vi "BuildThermomechanicalStave-Old.vi"() -> ()   [LabVIEW 2016] (continued)
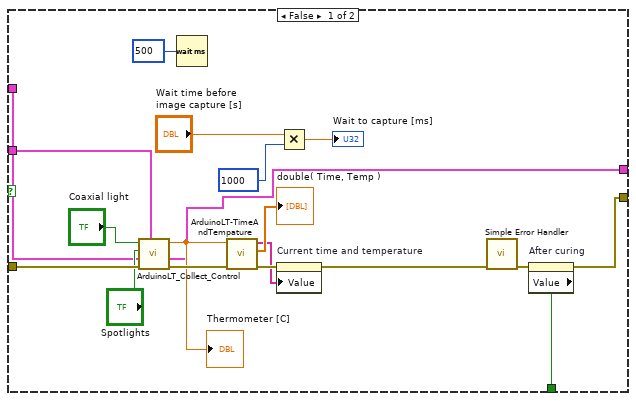
[diagram p3: hidden frame]
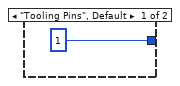
[diagram p4: hidden frame]
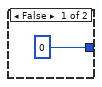
[diagram p5: hidden frame]
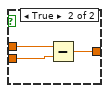
[diagram p9: hidden frame]
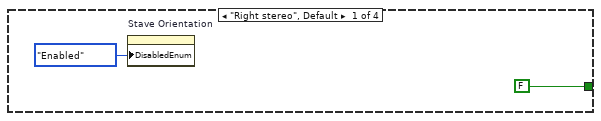
[diagram p10: hidden frame]
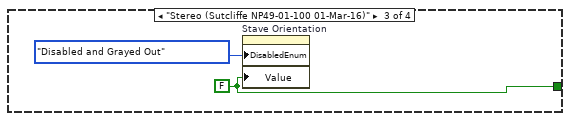
[diagram p11: hidden frame]
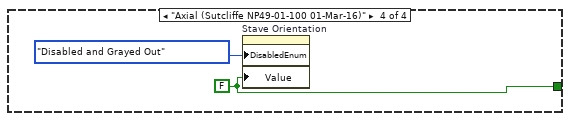
[diagram p12: hidden frame]
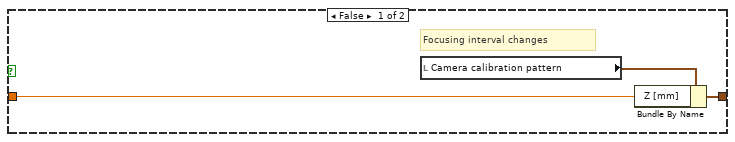
[diagram p16: hidden frame]
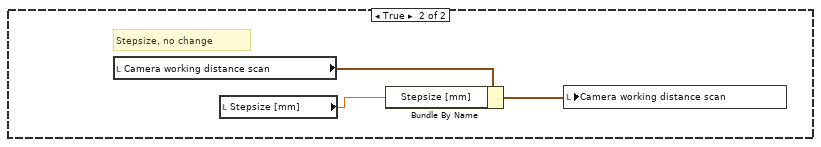
[diagram p17: hidden frame]
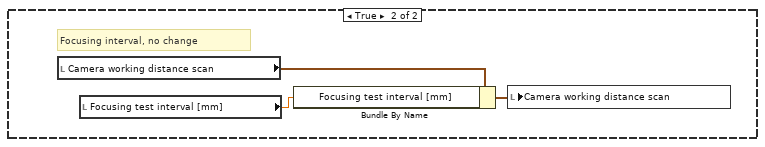
[diagram p18: hidden frame]
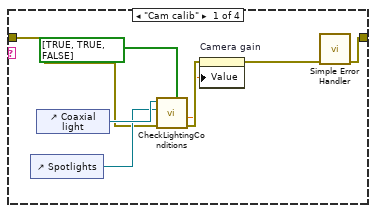
[diagram p19: hidden frame]
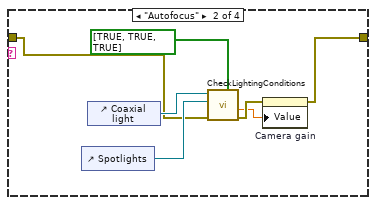
[diagram p20: hidden frame]
      n159 = Unbundle By Name("Jogging Controls") -> ("Jog step size"=w461:T16)
      n160 = control-ref of="Left"() -> (w468:refnum<vi>)
      n161 = control-ref of="Forward"() -> (w457:refnum<vi>)
      n162 = control-ref of="Up"() -> (w459:refnum<vi>)
      n163 = control-ref of="Right"() -> (w467:refnum<vi>)
      n164 = control-ref of="Backward"() -> (w456:refnum<vi>)
      n165 = call "JogStepInterpeter (SubVI).vi"("Jog step size ENUM"=w461) -> ("Jog step size"=w460:T37)
      n166 = call "ActivateToggleControls (SubVI).vi"("Left refnum"=w468, "Current stage position [mm]"=w464, "Right refnum"=w467, "Forward refnum"=w457, "Backward refnum"=w456, "error in (no error)"=w462, "Jog step size"=w460, "Up refnum"=w459, "Down refnum"=w458) -> ("error out"=w466:errorcluster)  [unwired: 6 in]
      n167 = event shown="[6] \"Jogging Controls.Confirm position\": Value Change" {
        selector: _ -> [_ _ _ _ _ _ _]
        dyn-events: _ -> [_ _ _ _ _ _ _]
        timeout: _ -> [_ _ _ _ _ _ _]
        tunnel: w475 -> [w482 w491 w496 w502 w506 w511 w522]
        tunnel: w466 -> [w481 w490 w495 w501 w505 w510 w520]
        tunnel: [w479 w489 w494 w499 w504 w509 w514] -> w471
        tunnel: [_ _ _ _ _ _ TRUE] -> w472
        tunnel: [w478 w488 w493 w498 w503 w508 w518] -> w470
        tunnel: [_ _ _ _ _ _ w513] -> w469
        tunnel: w460 -> [w477 _ _ _ _ _ _]
        tunnel: w464 -> [w476 _ _ _ _ _ _]
        event Timeout {
          n168 = event-data() -> ()  [unwired: 1 in, 2 out]
          n169 = control-ref of="Forward"() -> (w487:refnum<vi>)
          n170 = control-ref of="Left"() -> (w484:refnum<vi>)
          n171 = control-ref of="Right"() -> (w485:refnum<vi>)
          n172 = control-ref of="Backward"() -> (w486:refnum<vi>)
          n173 = call "ActivateToggleControls (SubVI).vi"("Left refnum"=w484, "Current stage position [mm]"=w476, "Right refnum"=w485, "Forward refnum"=w486, "Backward refnum"=w487, "error in (no error)"=w481, "Jog step size"=w477) -> ("error out"=w480:errorcluster)  [unwired: 8 in]
          n174 = Enqueue Element(queue=w482, element="NULL", error in (no error)=w480) -> (queue out=w478:refnum<queue>, error out=w479:errorcluster)  [unwired: 1 in, 1 out]
        }
        event Value Change {
          n175 = event-data() -> ()  [unwired: 1 in, 3 out]
          n176 = Enqueue Element(queue=w491, element="-X", error in (no error)=w490) -> (queue out=w488:refnum<queue>, error out=w489:errorcluster)  [unwired: 1 in, 1 out]
        }
        event Value Change {
          n177 = event-data() -> ()  [unwired: 1 in, 3 out]
          n178 = Enqueue Element(queue=w496, element="X", error in (no error)=w495) -> (queue out=w493:refnum<queue>, error out=w494:errorcluster)  [unwired: 1 in, 1 out]
        }
        event Value Change {
          n179 = event-data() -> ()  [unwired: 1 in, 3 out]
          n180 = Enqueue Element(queue=w502, element="Y", error in (no error)=w501) -> (queue out=w498:refnum<queue>, error out=w499:errorcluster)  [unwired: 1 in, 1 out]
        }
        event Value Change {
          n181 = event-data() -> ()  [unwired: 1 in, 3 out]
          n182 = Enqueue Element(queue=w506, element="-Y", error in (no error)=w505) -> (queue out=w503:refnum<queue>, error out=w504:errorcluster)  [unwired: 1 in, 1 out]
        }
        event Value Change {
          n183 = event-data() -> ()  [unwired: 1 in, 3 out]
          n184 = Enqueue Element(queue=w511, element="ALL", error in (no error)=w510) -> (queue out=w508:refnum<queue>, error out=w509:errorcluster)  [unwired: 1 in, 1 out]
        }
        event Value Change {
          n185 = event-data() -> ()  [unwired: 1 in, 3 out]
          n186 = Enqueue Element(queue=w522, element="DONE", error in (no error)=w520) -> (queue out=w518:refnum<queue>, error out=w517:errorcluster)  [unwired: 1 in, 1 out]
          n187 = property on="Confirm position" class="Bool (strict)"(error in=w517, "Value"=FALSE ("Confirm position")) -> (error out=w515:errorcluster)  [unwired: 1 in, 1 out]
          n188 = property on="Current stage position [mm]" class="Clust (strict)"(error in=w515) -> (error out=w514:errorcluster, "Value"=w513:cluster{"X":dbl, "Y":dbl, "Z":dbl})  [unwired: 1 in, 1 out]
        }
      }
      n189 = Unbundle By Name(w471) -> ("status"=w474:bool)
      n190 = Or(x=w474, y=w472) -> (x .or. y?=w473:bool)
    }
    n191 = Release Queue(queue=w358, error in (no error)=w357) -> (error out=w353:errorcluster)  [unwired: 1 in, 2 out]
  }
  n192 = call <vilib>:"Close.vi"("Arduino Resource"=w18, "error in"=w17) -> ("error out"=w16:errorcluster)  [unwired: 13 in]
  n193 = local write "VISA error out"(w16) -> ()
  n194 = Unbundle(w108) -> ("Camera session out"=w107:T8, "New Image"=w106:T23)
  n195 = Release Queue(queue=w110, error in (no error)=w109) -> (error out=w104:errorcluster)  [unwired: 1 in, 2 out]
  n196 = call "IMAQ Dispose"("Image"=w106, "error in (no error)"=w104) -> ("error out"=w105:errorcluster)  [unwired: 4 in]
  n197 = call <vilib>:"IMAQdx Close Camera.vi"("error in"=w105, "Session In"=w107) -> ("error out"=w102:errorcluster)  [unwired: 9 in]
  n198 = local write "Camera error out"(w102) -> ()
  n199 = call "File Dialog"("start path"="Reports path", "prompt"="Select reporting path") -> ("selected path"=w1:path)  [unwired: 10 in, 3 out]
  n200 = local write "Reports path"(w1) -> ()
  n201 = local write "Module fiducials in the XYZ stage's basis"(T2 [{"Generated List of Module Coordinates"=[], "Generated List of Module Coordinates"=[]}, {"Generated List of Module Coordinates"=[-299.2110287057527, -202.7315011933668, -202.42767808647434, -298.9072055988603, -201.21150863720152, -104.73198112481558, -104.42815801792312, -200.90768553030907, -103.2119885686503, -6.732461056264299, -6.4286379493718755, -102.90816546175785, -5.212468500099078, 91.2670590122869, 91.57088211917932, -4.908645393206655, 92.78705156845217, 189.26657908083814, 189.57040218773056, 93.0908746753446, 190.7865716370033, 287.2660991493893, 287.5699222562817, 191.09039474389573, 288.7860917055545, 385.26561921794047, 385.5694423248329, 289.0899148124469, 386.7856117741057, 483.26513928649166, 483.5689623933841, 387.0894348809981, 484.7851318426569, 581.2646593550428, 581.5684824619352, 485.0889549495493, 582.7846519112081, 679.264179423594, 679.5680025304864, 583.0884750181006, 680.7841719797593, 777.2636994921454, 777.5675225990378, 681.0879950866517, 778.7836920483107, 875.2632195606966, 875.567042667589, 779.0875151552032, 876.7832121168619, 973.2627396292478, 973.5665627361402, 877.0870352237544], "Generated List of Module Coordinates"=[18.614201133837582, 18.312255796456228, 115.39178037048637, 115.69372570786773, 18.307498780361485, 18.00555344298013, 115.08507801701028, 115.38702335439163, 18.0007964268854, 17.698851089504046, 114.77837566353418, 115.08032100091555, 17.694094073409303, 17.39214873602795, 114.4716733100581, 114.77361864743946, 17.38739171993322, 17.08544638255185, 114.16497095658201, 114.46691629396337, 17.080689366457122, 16.778744029075767, 113.85826860310591, 114.16021394048727, 16.77398701298104, 16.47204167559967, 113.55156624962981, 113.85351158701118, 16.46728465950494, 16.165339322123586, 113.24486389615373, 113.54680923353509, 16.160582306028857, 15.858636968647488, 112.93816154267763, 113.240106880059, 15.85387995255276, 15.551934615171405, 112.63145918920155, 112.9334045265829, 15.547177599076676, 15.245232261695307, 112.32475683572545, 112.62670217310682, 15.240475245600578, 14.938529908219223, 112.01805448224937, 112.31999981963072, 14.933772892124495, 14.631827554743126, 111.71135212877327, 112.01329746615463]}, {"Generated List of Module Coordinates"=[-250.8193533961135, -152.81983332756232, -54.82031325901109, 43.17920680954012, 141.17872687809137, 239.1782469466425, 337.1777670151937, 435.1772870837449, 533.1768071522961, 631.1763272208473, 729.1758472893986, 827.1753673579499, 925.1748874265011], "Generated List of Module Coordinates"=[67.00299075216198, 66.69628839868588, 66.3895860452098, 66.0828836917337, 65.77618133825762, 65.46947898478152, 65.16277663130543, 64.85607427782934, 64.54937192435324, 64.24266957087715, 63.935967217401064, 63.62926486392497, 63.32256251044888]}] ("Module fiducials in the XYZ stage's basis")) -> ()
  n202 = local read "XYZ Stage Frame: Coordinates for calibration"() -> (w156:T12)
  n203 = Array To Cluster(array=w158) -> (cluster=w157:T38)
  n204 = Merge Errors(w155) -> (w154:errorcluster)
  n205 = property on="Jog step size" class="Clust (strict)"(error in=w154, "DisabledEnum"=w49) -> (error out=w153:errorcluster)  [unwired: 1 in, 1 out]
  n206 = Unbundle By Name(w157) -> ("[0]"=w65:cluster{"X":dbl, "Y":dbl, "Z":dbl}, "[1]"=w147:cluster{"X":dbl, "Y":dbl, "Z":dbl}, "[2]"=w64:cluster{"X":dbl, "Y":dbl, "Z":dbl})
  "Stave origin" <- w65
  "Camera calibration pattern" <- w147
  "Bus tape circle" <- w64
  n207 = Bundle By Name(cluster=w156, "Stave Origin"=w65, "Cam calib"=w147, "Bus Tape Circle"=w64) -> (w152:T12)
  n208 = Unbundle By Name(w147) -> ("Z"=→"Baseline Z [mm]":dbl)
  n209 = property on="Left" class="Bool (strict)"(error in=w153, "DisabledEnum"=w49, "Value"=w50) -> (error out=w48:errorcluster)  [unwired: 1 in, 1 out]
  n210 = property on="Up" class="Bool (strict)"(error in=w48, "DisabledEnum"=w49, "Value"=w50) -> (error out=w47:errorcluster)  [unwired: 1 in, 1 out]
  n211 = property on="Down" class="Bool (strict)"(error in=w48, "DisabledEnum"=w49, "Value"=w50) -> (error out=w46:errorcluster)  [unwired: 1 in, 1 out]
  n212 = property on="Current Build Phase" class="Str"(error in=w48, "Value"="Preparing to calibrate camera height...") -> (error out=w140:errorcluster)  [unwired: 1 in, 1 out]
  n213 = property on="Confirm position" class="Bool (strict)"(error in=w48, "DisabledEnum"=w49, "Value"=w50) -> (error out=w139:errorcluster)  [unwired: 1 in, 1 out]
  n214 = property on="Reset position" class="Bool (strict)"(error in=w48, "DisabledEnum"=w49, "Value"=w50) -> (error out=w138:errorcluster)  [unwired: 1 in, 1 out]
  n215 = property on="Forward" class="Bool (strict)"(error in=w48, "DisabledEnum"=w49, "Value"=w50) -> (error out=w137:errorcluster)  [unwired: 1 in, 1 out]
  n216 = property on="Backward" class="Bool (strict)"(error in=w48, "DisabledEnum"=w49, "Value"=w50) -> (error out=w136:errorcluster)  [unwired: 1 in, 1 out]
  n217 = property on="Right" class="Bool (strict)"(error in=w48, "DisabledEnum"=w49, "Value"=w50) -> (error out=w135:errorcluster)  [unwired: 1 in, 1 out]
  n218 = property on="XYZ Stage Frame: Coordinates for calibration" class="Clust (strict)"(error in=w48, "Value"=w152) -> (error out=w134:errorcluster)  [unwired: 1 in, 1 out]
  n219 = control-ref of="Spotlights"() -> (w32:refnum<vi>)
  n220 = control-ref of="Coaxial light"() -> (w33:refnum<vi>)
  n221 = Merge Errors(w140, w139, w138, w137, w136, w135, w134, w47, w46) -> (w31:errorcluster)
  n222 = call "CheckLightingConditions.vi"("Change Lights? (Change; Coax; Spotlight)"=bool[] [TRUE, TRUE, FALSE], "error in (no error)"=w31, "Spotlights Refnum"=w32, "Coaxial Lights Refnum"=w33) -> ("error out"=w30:errorcluster, "Assigned Camera Gain"=w29:dbl)  [unwired: 4 in, 2 out]
  "Camera Gain Autofocus" <- w29
  n223 = property on="Camera gain" class="DigNum (strict)"(error in=w30, "Value"=w29) -> (error out=w150:errorcluster)  [unwired: 1 in, 1 out]
  n224 = while "CALIBRATE CAMERA  (AUTOFOCUSING AND PIX-UM CONVERSION)" {
    shift-right: [w554] -> w161
    shift-left: w150 -> [w557]
    tunnel: w100 -> [w566]
    tunnel: [w565] -> w99
    tunnel: [w558] -> w63
    tunnel: [w534] -> w66
    i -> [w563]
    stop <- w551 stop-if-true
    w526 = T40 1 items=["Strip Centers", "Signal Fit, Left to Right", "Projection + Signal Fit"] ("um/pix conversion method")
    # "update central value, stepsize, focusing test interval"
    n225 = local read "Camera Gain Autofocus"() -> (w552:dbl)
    n226 = local read "Reports path"() -> (w523:path)
    n227 = Unbundle By Name("Camera working distance scan") -> ("Stepsize [mm]"=w545:dbl, "Focusing test interval [mm]"=w544:dbl)
    "Stepsize [mm]" <- w545
    "Focusing test interval [mm]" <- w544
    n228 = property on="Camera gain" class="DigNum (strict)"(error in=w557, "Value"=w552) -> (error out=w556:errorcluster)  [unwired: 1 in, 1 out]
    n229 = Build Path(base path=w523, name or relative path="cameracalib") -> (appended path=w562:path)
    n230 = local read "Camera calibration pattern"() -> (w549:T25)
    n231 = Multiply(x=w544, y=2.0) -> (x*y=w546:dbl)
    n232 = Divide(x=w546, y=w545) -> (x/y=w547:dbl)
    n233 = call "RecursiveDirectoryStructureGenerator (SubVI).vi"("error in (no error)"=w556, "Folder index"=w563, "Host directory"=w562) -> ("error out"=w564:errorcluster, "Nth subfolder in host directory"=w539:path)  [unwired: 7 in]
    n234 = for {
      N: w547 -> [_]
      tunnel: w549 -> [w591]
      tunnel: [w588] -> w543 mode=indexing
      tunnel: w545 -> [w586]
      tunnel: w544 -> [w581]
      i -> [w587]
      n235 = Unbundle By Name(w591) -> ("X [mm]"=w590:dbl, "Y [mm]"=w589:dbl, "Z [mm]"=w585:dbl)
      n236 = local write "Image Collection Progress"(u8 0 ("Image Collection Status")) -> ()
      n237 = Subtract(x=w585, y=w581) -> (x-y=w584:dbl)
      n238 = Multiply(x=w586, y=w587) -> (x*y=w583:dbl)
      n239 = Add(x=w584, y=w583) -> (x+y=w582:dbl)
      n240 = Build Array(w590, w589, w582) -> (w588:dbl[])
    }
    n241 = property on="Axis Speeds [mm/s]" class="Clust (strict)"(error in=w564) -> (error out=w530:errorcluster, "Value"=w567:cluster{"X":dbl, "Y":dbl, "Z":dbl})  [unwired: 1 in, 1 out]
    n242 = local read "Current field of view"() -> (w573:T23)
    n243 = local read "double( Time, Temp )"() -> (w542:dbl[])
    n244 = property on="Current Build Phase" class="Str"(error in=w530, "Value"="Collecting images to calibrate camera..." ("Current Build Phase")) -> (error out=w531:errorcluster)  [unwired: 1 in, 1 out]
    n245 = Bundle("Current field of view"=w573, "Value"=w567, "Aerotech out"=w566) -> (w550:T41)  [unwired: 1 in]
    "Image collection inputs" <- w550
    n246 = local read "Wait to capture [ms]"() -> (w541:u32)
    n247 = local read "Calibration Results"() -> (w575:T14)
    n248 = control-ref of="Image Collection Progress"() -> (w525:refnum<vi>)
    n249 = call "CollectImageSet (SubVI).vi"("Inputs"=w550, "Path to save collected images"=w539, "milliseconds to wait"=w541, "Set of coordinates to process"=w543, "Time & Temperature Stamp"=w542, "error in"=w531, "Image Collection Refnum"=w525) -> ("Outputs"=w540:T42, "error out"=w529:errorcluster)  [unwired: 6 in, 1 out]
    n250 = property on="Current Build Phase" class="Str"(error in=w529, "Value"="Finding optimal height and pix-micron connversion..." ("Current Build Phase")) -> (error out=w528:errorcluster)  [unwired: 1 in, 1 out]
    n251 = local read "Strip pitch [um]"() -> (w524:dbl)
    n252 = call "1_2_UnifiedCameraCalibration.vi"("um/pix conversion method"=w526, "Sharpness assessment method"=Enum_TypeDef_ImageSharpnessAnalysisMethod."Mean( Laplacian Convolution )", "error in (no error)"=w528, "Strip Pitch (microns)"=w524, "Naming Convention"="*.png", "Images Directory"=w539) -> ("error out"=w535:errorcluster, "Camera calibration results"=w537:T13)  [unwired: 4 in]
    n253 = Bundle By Name(cluster=w575, "Camera calibration results"=w537) -> (w570:T14)
    n254 = Unbundle By Name(w537) -> ("Working distance to stave [mm]"=w534:dbl, "Calibration [um/pix]"=→"Average microns/pixel":dbl)
    "Optimized Z [mm]" <- w534
    n255 = local read "Baseline Z [mm]"() -> (w574:dbl)
    n256 = Subtract(x=w574, y=w534) -> (x-y=→"delta Z":dbl)
    n257 = property on="Calibration Results" class="Clust (strict)"(error in=w535, "Value"=w570) -> (error out=w569:errorcluster)  [unwired: 1 in, 1 out]
    n258 = call <vilib>:"Simple Error Handler.vi"("error in (no error)"=w569) -> ("error out"=w568:errorcluster)  [unwired: 4 in, 4 out]
    n259 = call "Accept camera working distance?"("error in (no error)"=w568) -> ("Gain"=w553:dbl, "Update focusing test interval [mm]"=w559:dbl, "Update stepsize [mm]"=w560:dbl, "Update central value [mm]"=w561:dbl, "Accept calibration"=w551:bool, "error out"=w555:errorcluster)  [unwired: 12 in, 1 out]
    n260 = property on="Camera gain" class="DigNum (strict)"(error in=w555, "Value"=w553) -> (error out=w554:errorcluster)  [unwired: 1 in, 1 out]
    n261 = local write "Camera Gain Autofocus"(w553) -> ()
    n262 = Equal To 0?(x=w560) -> (x = 0?=w578:bool)
    n263 = Equal To 0?(x=w559) -> (x = 0?=w579:bool)
    n264 = Equal To 0?(x=w561) -> (x = 0?=w577:bool)
    n265 = case shown="False" w578 {
      tunnel: w560 -> [w600 _]
      tunnel: w560 -> [w599 _]
      frame False {
        # "Stepsize changes"
        n266 = local write "Stepsize [mm]"(w599) -> ()
        n267 = local read "Camera working distance scan"() -> (w601:T11)
        n268 = Bundle By Name(cluster=w601, "Stepsize [mm]"=w600) -> (w602:T11)
        n269 = local write "Camera working distance scan"(w602) -> ()
      }
      frame True {
        # "Stepsize, no change"
        n270 = local read "Camera working distance scan"() -> (w604:T11)
        n271 = local read "Stepsize [mm]"() -> (w603:dbl)
        n272 = Bundle By Name(cluster=w604, "Stepsize [mm]"=w603) -> (w605:T11)
        n273 = local write "Camera working distance scan"(w605) -> ()
      }
    }
    n274 = case shown="False" w579 {
      tunnel: w559 -> [w607 _]
      tunnel: w559 -> [w606 _]
      frame False {
        # "Focusing interval changes"
        n275 = local write "Focusing test interval [mm]"(w606) -> ()
        n276 = local read "Camera working distance scan"() -> (w608:T11)
        n277 = Bundle By Name(cluster=w608, "Focusing test interval [mm]"=w607) -> (w609:T11)
        n278 = local write "Camera working distance scan"(w609) -> ()
      }
      frame True {
        # "Focusing interval, no change"
        n279 = local read "Camera working distance scan"() -> (w611:T11)
        n280 = local read "Focusing test interval [mm]"() -> (w610:dbl)
        n281 = Bundle By Name(cluster=w611, "Focusing test interval [mm]"=w610) -> (w612:T11)
        n282 = local write "Camera working distance scan"(w612) -> ()
      }
    }
    n283 = case shown="True" w577 {
      tunnel: w561 -> [w593 _]
      tunnel: [w592 w595] -> w558
      frame False {
        # "Focusing interval changes"
        n284 = local read "Camera calibration pattern"() -> (w594:T25)
        n285 = Bundle By Name(cluster=w594, "Z [mm]"=w593) -> (w592:T25)
      }
      frame True {
        # "Central value, no change"
        n286 = local read "Camera calibration pattern"() -> (w597:T25)
        n287 = local read "Camera calibration pattern"() -> (w598:T25)
        n288 = Unbundle By Name(w597) -> ("Z [mm]"=w596:dbl)
        n289 = Bundle By Name(cluster=w598, "Z [mm]"=w596) -> (w595:T25)
      }
    }
    n290 = Unbundle By Name(w540) -> ("XYZ .NET Refnum out"=w565:refnum<k24>)
    n291 = local write "Camera calibration pattern"(w558) -> ()
  }
  "Calibrated module height" <- w66
  n292 = Bundle By Name(cluster="XYZ Stage Frame: Coordinates for calibration", "Cam calib"=w63) -> (w61:T12)
  n293 = property on="Camera height" class="Bool (strict)"(error in=w161, "Value"=TRUE) -> (error out=w160:errorcluster)  [unwired: 1 in, 1 out]
  n294 = property on="Tape Type" class="Enum (strict)"() -> ("Value"=w77:T5)  [unwired: 2 in, 2 out]
  n295 = property on="XYZ Stage Frame: Coordinates for calibration" class="Clust (strict)"(error in=w160, "Value"=w61) -> (error out=w24:errorcluster)  [unwired: 1 in, 1 out]
  n296 = Unbundle By Name(w61) -> ("Bus Tape Circle"=w58:T25, "Stave Origin"=w60:T25)
  n297 = case "Visualize stave orientation" shown="\"Left stereo\"" w77 {
    tunnel: [FALSE w615 w617 w619] -> w76
    frame "Right stereo", Default {
      n298 = property on="Stave Orientation" class="Bool"("DisabledEnum"=T27."Enabled" ("Disabled")) -> ()  [unwired: 2 in, 2 out]
    }
    frame "Left stereo" {
      w615 = TRUE
      n299 = property on="Stave Orientation" class="Bool"("DisabledEnum"=T27."Enabled" ("Disabled"), "Value"=w615) -> ()  [unwired: 2 in, 2 out]
    }
    frame "Stereo (Sutcliffe NP49-01-100 01-Mar-16)" {
      w617 = FALSE
      n300 = property on="Stave Orientation" class="Bool"("DisabledEnum"=T27."Disabled and Grayed Out" ("Disabled"), "Value"=w617) -> ()  [unwired: 2 in, 2 out]
    }
    frame "Axial (Sutcliffe NP49-01-100 01-Mar-16)" {
      w619 = FALSE
      n301 = property on="Stave Orientation" class="Bool"("DisabledEnum"=T27."Disabled and Grayed Out" ("Disabled"), "Value"=w619) -> ()  [unwired: 2 in, 2 out]
    }
  }
  "Stave Orientation" <- w76
  n302 = control-ref of="Spotlights"() -> (w35:refnum<vi>)
  n303 = control-ref of="Coaxial light"() -> (w34:refnum<vi>)
  n304 = Build Path(base path=w1, name or relative path="staveCalib") -> (appended path=w174:path)
  n305 = disable-structure shown="Disabled" {
    frame Disabled {
      n306 = local read "delta Z"() -> ()  [unwired: 1 out]
    }
    frame Enabled {
    }
  }
  n307 = call "CheckLightingConditions.vi"("Change Lights? (Change; Coax; Spotlight)"=bool[] [TRUE, TRUE, TRUE], "error in (no error)"=w24, "Spotlights Refnum"=w35, "Coaxial Lights Refnum"=w34) -> ("error out"=w26:errorcluster, "Assigned Camera Gain"=w25:dbl)  [unwired: 4 in, 2 out]
  n308 = property on="Stave Coordinate System" class="Enum (strict)"(error in=w24) -> (error out=w125:errorcluster, "Value"=w68:enum16{"Tooling Pins", "Bus Tape"})  [unwired: 1 in, 1 out]
  n309 = property on="Current Build Phase" class="Str"(error in=w24, "Value"="Locating locking points..." ("Current Build Phase")) -> (error out=w121:errorcluster)  [unwired: 1 in, 1 out]
  n310 = call <vilib>:"Check if File or Folder Exists.vi"("error in (no error)"=w24, "path"=w174) -> ("error out"=w173:errorcluster, "file or folder exists?"=w175:bool)  [unwired: 7 in, 1 out]
  n311 = Unbundle By Name(w58) -> ("X [mm]"=w55:dbl, "Y [mm]"=w56:dbl, "Z [mm]"=w59:dbl)
  n312 = case shown="True" w175 {
    tunnel: w174 -> [w624 w626]
    tunnel: [w623 w626] -> w172
    tunnel: w173 -> [w622 w625]
    tunnel: [w621 w625] -> w123
    frame False {
      n313 = Create Folder(path (use dialog)=w624, error in=w622) -> (created path=w623:path, error out=w621:errorcluster)  [unwired: 1 in, 1 out]
    }
    frame True {
    }
  }
  n314 = property on="Axis Speeds [mm/s]" class="Clust (strict)"(error in=w24) -> (error out=w124:errorcluster, "Value"=w145:cluster{"X":dbl, "Y":dbl, "Z":dbl})  [unwired: 1 in, 1 out]
  n315 = property on="Pix/um" class="Bool (strict)"(error in=w24, "Value"=TRUE) -> (error out=w122:errorcluster)  [unwired: 1 in, 1 out]
  n316 = property on="Camera gain" class="DigNum (strict)"(error in=w26, "Value"=w25) -> (error out=w120:errorcluster)  [unwired: 1 in, 1 out]
  n317 = Unbundle By Name(w60) -> ("X [mm]"=w169:dbl, "Y [mm]"=w170:dbl, "Z [mm]"=w168:dbl)
  n318 = local read "delta Z"() -> (w62:dbl)
  n319 = local read "Code path"() -> (w166:path)
  n320 = Add(x=w59, y=w62) -> (x+y=w57:dbl)
  n321 = Add(x=w168, y=0.0) -> (x+y=w171:dbl)
  n322 = local read "double( Time, Temp )"() -> (w79:dbl[])
  n323 = local read "Wait to capture [ms]"() -> (w163:u32)
  n324 = case shown="\"Bus Tape\"" w68 {
    tunnel: [1 w629] -> w67
    frame "Tooling Pins", Default {
    }
    frame "Bus Tape" {
      n325 = case shown="True" "Quick Calib?" {
        tunnel: [0 2] -> w629
        frame False {
        }
        frame True {
        }
      }
    }
  }
  "Calibration Type" <- w67
  n326 = Bundle By Name(cluster=w60, "X [mm]"=w169, "Y [mm]"=w170, "Z [mm]"=w171) -> (w167:T25)
  n327 = Bundle By Name(cluster=w58, "X [mm]"=w55, "Y [mm]"=w56, "Z [mm]"=w57) -> (w54:T25)
  n328 = Merge Errors(w123, w125, w124, w122, w121, w120) -> (w126:errorcluster)
  n329 = Build Path(base path=w166, name or relative path="Utils\\ConfigurationFiles_and_Templates\\0_Calibration") -> (appended path=w164:path)
  n330 = while {
    tunnel: 2 ("N pics captured") -> [w728]
    tunnel: w172 -> [w726]
    tunnel: w167 -> [w725]
    tunnel: w164 -> [w723]
    tunnel: w163 -> [w721]
    tunnel: [w632] -> _
    tunnel: w145 -> [w706]
    tunnel: w68 -> [w705]
    tunnel: w126 -> [w643]
    tunnel: w79 -> [w688]
    tunnel: w54 -> [w687]
    tunnel: w76 -> [w683]
    tunnel: [w653] -> w71
    tunnel: [w656] -> w69
    shift-right: [w657] -> w70
    shift-left: w99 -> [w692]
    stop <- w655 stop-if-true
    (unwired) dbl[] [-19.597, -9.7121] ("y")
    (unwired) dbl[] [58.39, 9.7121] ("y")
    (unwired) dbl[] [-184.207, 10.734] ("y")
    (unwired) dbl[] [-184.391, 9.908] ("y")
    # "Module centres, in the stave basis >>"
    # "Fiducials, in the stave basis >>"
    # "User must confirm coordinates to proceed"
    # "import contents of visually inspect list of coordinates\nso that they display on the front panel"
    n331 = local read "Current field of view"() -> (w632:T23)
    n332 = control-ref of="Spotlights"() -> (w646:refnum<vi>)
    n333 = control-ref of="Coaxial light"() -> (w645:refnum<vi>)
    n334 = call "CheckLightingConditions.vi"("Change Lights? (Change; Coax; Spotlight)"=bool[] [TRUE, TRUE, TRUE], "error in (no error)"=w643, "Spotlights Refnum"=w646, "Coaxial Lights Refnum"=w645) -> ("error out"=w642:errorcluster, "Assigned Camera Gain"=w641:dbl)  [unwired: 4 in, 2 out]
    n335 = local read "Average microns/pixel"() -> (w648:ext)
    n336 = control-ref of="Current Build Phase"() -> (w649:refnum<vi>)
    n337 = local read "Calibration Type"() -> (w652:u16)
    n338 = property on="Camera gain" class="DigNum (strict)"(error in=w642, "Value"=w641) -> (error out=w650:errorcluster)  [unwired: 1 in, 1 out]
    n339 = control-ref of="Image Collection Progress"() -> (w647:refnum<vi>)
    n340 = control-ref of="Calibration Results"() -> (w722:refnum<vi>)
    n341 = call "0_StageToStave.vi"("Image feed"=w632, "Stave origin in XYZ Frame"=w725, "Stave Coordinate System"=w705, "Pixel resolution [um/pix]"=w648, "Axes Speeds [mm/s]"=w706, "Number of pictures at each point"=w728, "Pause before image capture [ms]"=w721, "Error in"=w650, "Time & Temperature Stamp"=w688, "Record keeping file path"=w726, "Stave Orientation"=w683, "XYZ .NET Refnum in"=w692, "Autofocus Coord in XYZ Frame"=w687, "Current Build Phase"=w649, "Templates path"=w723, "Image Collection Refnum"=w647, "Calibration Type"=w652, "Calibration Results"=w722) -> ("Cross- check: Are these the center of pins in the center of the image?"=w727:T23[], "XYZ .NET Refnum out"=w691:refnum<k24>, "Angle of stave  [rad]"=w673:dbl, "Calibrated stave origin (X,Y) [mm]"=w674:dbl[], "Calibrated stave basis [mm]"=→"Calibrated stave basis [mm]":dbl[][], "Error out"=w663:errorcluster)  [unwired: 3 in, 1 out]
    "Angle between stave and xyz stage" <- w673
    "Calibrated stave origin (X,Y) [mm]" <- w674
    n342 = local read "Reports path"() -> (w682:path)
    n343 = call "Prompt User for Input"("error in (no error)"=w663) -> ("Notes"=w676:string, "Stave ID"=w677:string, "OK"=w680:bool, "error out"=w681:errorcluster)  [unwired: 15 in]
    "Stave ID" <- w677
    n344 = call "DumpImageSet (SubVI).vi"("error in (no error)"=w663, "Calibrated Image Array"=w727) -> ("error out"=w678:errorcluster)  [unwired: 6 in]
    n345 = local read "Optimized Z [mm]"() -> (w672:dbl)
    n346 = Build Path(base path=w682, name or relative path="CalibrationResults.ini") -> (appended path=w675:path)
    n347 = call "WriteCalibrationToFile (SubVI).vi"("Stave ID"=w677, "User notes"=w676, "CameraWD"=w672, "um/Pixel"=w648, "Angle"=w673, "Stave Origin"=w674, "error in (no error)"=w681, "Calibration file path"=w675, "Write to file"=w680) -> ("error out"=w671:errorcluster)  [unwired: 10 in]
    n348 = Merge Errors(w671, w678) -> (w697:errorcluster)
    n349 = property on="Current Build Phase" class="Str"(error in=w697, "Value"="Fetching the virtual stave..." ("Current Build Phase")) -> (error out=w693:errorcluster)  [unwired: 1 in, 1 out]
    n350 = property on="Stave basis" class="Bool (strict)"(error in=w697, "Value"=TRUE) -> (error out=w694:errorcluster)  [unwired: 1 in, 1 out]
    n351 = property on="Calibrated?" class="Clust (strict)"(error in=w697, "Color"=u32 1089280) -> (error out=w695:errorcluster)  [unwired: 1 in, 1 out]
    n352 = control-ref of="Spotlights"() -> (w640:refnum<vi>)
    n353 = control-ref of="Coaxial light"() -> (w639:refnum<vi>)
    n354 = Merge Errors(w694, w695, w693) -> (w696:errorcluster)
    n355 = call <vilib>:"Simple Error Handler.vi"("error in (no error)"=w696) -> ("error out"=w636:errorcluster)  [unwired: 4 in, 4 out]
    n356 = call "CheckLightingConditions.vi"("Change Lights? (Change; Coax; Spotlight)"=bool[] [TRUE, TRUE, FALSE], "error in (no error)"=w636, "Spotlights Refnum"=w640, "Coaxial Lights Refnum"=w639) -> ("error out"=w637:errorcluster, "Assigned Camera Gain"=w635:dbl)  [unwired: 4 in, 2 out]
    n357 = property on="Camera gain" class="DigNum (strict)"(error in=w637, "Value"=w635) -> (error out=w712:errorcluster)  [unwired: 1 in, 1 out]
    n358 = local read "Calibrated module height"() -> (w734:dbl)
    n359 = Unbundle By Name("Build Config") -> ("Tape Type"=w684:T5, "Module fiducial marker"=w685:T7, "N Modules"=w689:i32)
    n360 = local read "Sensor Pattern"() -> (w633:T10)
    n361 = local read "Code path"() -> (w686:path)
    n362 = call "0_PlanVirtualStave.vi"("Tape Type"=w684, "Code path"=w686, "Module fiducial marker"=w685, "Sensor Pattern"=w633, "N Modules"=w689, "Working height [mm]"=w734, "error in (no error)"=w712) -> ("Stave Basis: Coordinates of Fiducials on Modules"=w737:dbl[][], "error out"=w736:errorcluster)  [unwired: 6 in, 1 out]
    n363 = property on="Tape Type" class="Enum (strict)"(error in=w736) -> (error out=w711:errorcluster, "Strings []"=w741:string[])  [unwired: 1 in, 1 out]
    n364 = Index Array(array=w741) -> (element=w739:string)  [unwired: 1 in]
    n365 = Concatenate Strings("Aligning real and virtual " ("Current Build Phase"), w739, " staves..." ("string")) -> (w729:string)
    n366 = property on="Current Build Phase" class="Str"(error in=w711, "Value"=w729) -> (error out=w710:errorcluster)  [unwired: 1 in, 1 out]
    n367 = for "Align real & virtual staves: (1) Rotate VS (2) Translate VS" {
      tunnel: w737 -> [w819] mode=indexing
      tunnel: [w816] -> w774 mode=indexing
      tunnel: w710 -> [w807]
      tunnel: [w806] -> w735 mode=indexing
      n368 = local read "Calibrated stave origin (X,Y) [mm]"() -> (w795:dbl[])
      n369 = Index Array(array=w819, index #1=0 ("index"), index #2=1 ("index"), index #3=2 ("index")) -> (element #1=w810:dbl, element #2=w785:dbl, element #3=w812:dbl)
      n370 = Negate(x=w785) -> (-x=w784:dbl)
      n371 = local read "Stave Orientation"() -> (w811:bool)
      n372 = local read "Angle between stave and xyz stage"() -> (w809:dbl)
      n373 = Index Array(array=w795, index #1=0 ("index"), index #2=1 ("index")) -> (element #1=w805:dbl, element #2=w804:dbl)
      n374 = Add(x=w804, y=w784) -> (x+y=w799:dbl)
      n375 = case shown="False" w811 {
        tunnel: [w826 w829] -> w802
        tunnel: w805 -> [w824 w827]
        tunnel: w810 -> [w825 w828]
        frame False {
          n376 = Add(x=w824, y=w825) -> (x+y=w826:dbl)
        }
        frame True {
          n377 = Subtract(x=w827, y=w828) -> (x-y=w829:dbl)
        }
      }
      n378 = Bundle(w805, w804) -> (w796:cluster{dbl, dbl})  [unwired: 1 in]
      n379 = Negate(x=w796) -> (-x=w803:cluster{dbl, dbl})
      n380 = call-poly <vilib>:"2D Cartesian Coordinate Shift.vi"("shift"=w803, "y"=w799, "x"=w802) -> ("y out"=w800:dbl, "x out"=w801:dbl)  [unwired: 6 in, 1 out]
      n381 = property on="Stave Coordinate System" class="Enum (strict)"() -> ("Value"=w794:enum16{"Tooling Pins", "Bus Tape"})  [unwired: 2 in, 2 out]
      n382 = call "RotateCoordinate (SubVI).vi"("Units"=enum16{"mrad", "Radians", "Degrees"}."Radians", "Angle"=w809, "error in (no error)"=w807, "y"=w800, "x"=w801) -> ("error out"=w806:errorcluster, "y'"=w797:dbl, "x'"=w798:dbl)  [unwired: 4 in]
      n383 = call-poly <vilib>:"2D Cartesian Coordinate Shift.vi"("shift"=w796, "y"=w797, "x"=w798) -> ("y out"=w792:dbl, "x out"=w793:dbl)  [unwired: 6 in, 1 out]
      n384 = Build Array(w793, w792) -> (w791:dbl[])
      n385 = case shown="\"Bus Tape\"" w794 {
        tunnel: [w820 w823] -> w790
        tunnel: w791 -> [w820 w822]
        frame "Tooling Pins", Default {
        }
        frame "Bus Tape" {
          n386 = Add(x=w822, y=dbl[] [-59.015, -10.1936]) -> (x+y=w823:dbl[])
        }
      }
      n387 = Index Array(array=w790, index #1=0 ("index"), index #2=1 ("index")) -> (element #1=w787:dbl, element #2=w786:dbl)
      n388 = Build Array(w787, w786, w812) -> (w816:dbl[])
    }
    n389 = local read "Reports path"() -> (w748:path)
    n390 = Merge Errors(w735) -> (w744:errorcluster)
    n391 = Build Path(base path=w748, name or relative path="virtualstave.csv") -> (appended path=w746:path)
    n392 = call-poly <vilib>:"Write Delimited Spreadsheet.vi"("file path (dialog if empty)"=w746, "format (%.3f)"="%.9f", "2D data"=w774, "error in (no error)"=w744, "delimiter (\\t)"="," ("delimiter (\\t)")) -> ("error out"=w742:errorcluster)  [unwired: 9 in, 1 out]
    n393 = property on="Tape Type" class="Enum (strict)"(error in=w742) -> (error out=w709:errorcluster, "Strings []"=w764:string[], "Value"=w699:T5)  [unwired: 1 in, 1 out]
    n394 = Index Array(array=w764, index=w699) -> (element=w766:string)
    n395 = Concatenate Strings("Preparing to position modules with " ("Current Build Phase"), w766, " stave coordinates..." ("string")) -> (w717:string)
    n396 = property on="Current Build Phase" class="Str"(error in=w709, "Value"=w717) -> (error out=w702:errorcluster)  [unwired: 1 in, 1 out]
    n397 = property on="N Modules" class="DigNum (strict)"(error in=w702) -> (error out=w703:errorcluster, "Value"=w704:i32)  [unwired: 1 in, 1 out]
    n398 = for {
      N: w704 -> [_]
      tunnel: w774 -> [w838]
      tunnel: [w833] -> w751 mode=indexing
      tunnel: [w832] -> w750 mode=indexing
      tunnel: w703 -> [w831]
      tunnel: [w830] -> w733 mode=indexing
      i -> [w837]
      w835 = 4 ("x")
      n399 = Multiply(x=w835, y=w837) -> (x*y=w836:i32)
      n400 = Array Subset(array=w838, index (row)=w836, length (row)=w835) -> (w834:dbl[][])  [unwired: 2 in]
      n401 = call "GetModuleCentre (SubVI).vi"("error in (no error)"=w831, "4x3 Array of Fiducial Coordinates"=w834) -> ("error out"=w830:errorcluster, "y, centre"=w832:dbl, "x, centre"=w833:dbl)  [unwired: 1 in]
    }
    n402 = local read "Calibrated stave basis [mm]"() -> (w752:dbl[][])
    n403 = Index Array(array=w774, index (col) #1=0 ("disabled index (col)"), index (col) #2=1 ("index (col)")) -> (element #1=w753:dbl[], element #2=w754:dbl[])  [unwired: 2 in]
    n404 = Index Array(array=w752, index (col) #1=0 ("disabled index (col)"), index (col) #2=1 ("disabled index (col)")) -> (element #1=w757:dbl[], element #2=w758:dbl[])  [unwired: 2 in]
    n405 = Bundle(w753, w754) -> (w761:cluster{dbl[], dbl[]})  [unwired: 1 in]
    n406 = Bundle("Calibrated stave basis [mm]"=w757, "Calibrated stave basis [mm]"=w758) -> (w762:T43)  [unwired: 1 in]
    n407 = Bundle(w751, w750) -> (w749:cluster{dbl[], dbl[]})  [unwired: 1 in]
    n408 = Merge Errors(w733) -> (w715:errorcluster)
    n409 = Build Array(w762, w761, w749) -> (→"Module fiducials in the XYZ stage's basis":T44)
    n410 = property on="Virtual stave" class="Bool (strict)"(error in=w715, "Value"=TRUE) -> (error out=w714:errorcluster)  [unwired: 1 in, 1 out]
    n411 = property on="Tape Type" class="Enum (strict)"(error in=w714) -> (error out=w708:errorcluster, "Strings []"=w732:string[], "Value"=w698:T5)  [unwired: 1 in, 1 out]
    n412 = local read "Stave ID"() -> (w659:string)
    n413 = Index Array(array=w732, index=w698) -> (element=w661:string)
    n414 = Concatenate Strings("Positioning modules on the " ("Current Build Phase"), w661, " side: Consult VisualizingModulePositions front panel... " ("Current Build Phase")) -> (w716:string)
    n415 = local read "Reports path"() -> (w668:path)
    n416 = property on="Current Build Phase" class="Str"(error in=w708, "Value"=w716) -> (error out=w666:errorcluster)  [unwired: 1 in, 1 out]
    n417 = Concatenate Strings("Stave: " ("string"), w659, ", Tape type: " ("string"), w661) -> (w658:string)
    n418 = Build Path(base path=w668, name or relative path="ModulePlacement") -> (appended path=w665:path)
    n419 = call <vilib>:"Check if File or Folder Exists.vi"("error in (no error)"=w666, "path"=w665) -> ("error out"=w669:errorcluster, "file or folder exists?"=w670:bool)  [unwired: 7 in, 1 out]
    n420 = local read "Average microns/pixel"() -> (w770:ext)
    n421 = control-ref of="Module Progress Report"() -> (w772:refnum<vi>)
    n422 = local read "Current field of view"() -> (w768:T23)
    n423 = case shown="False" w670 {
      tunnel: w665 -> [w781 w783]
      tunnel: [w778 w783] -> w664
      tunnel: w669 -> [w780 w782]
      tunnel: [w779 w782] -> w656
      frame False {
        n424 = Create Folder(path (use dialog)=w781, error in=w780) -> (created path=w778:path, error out=w779:errorcluster)  [unwired: 1 in, 1 out]
      }
      frame True {
      }
    }
    n425 = property on="Axis Speeds [mm/s]" class="Clust (strict)"(error in=w666) -> (error out=w700:errorcluster, "Value"=w701:cluster{"X":dbl, "Y":dbl, "Z":dbl})  [unwired: 1 in, 1 out]
    n426 = control-ref of="Processing module #"() -> (w707:refnum<vi>)
    n427 = control-ref of="Current Build Phase"() -> (w769:refnum<vi>)
    n428 = local read "Code path"() -> (w773:path)
    n429 = control-ref of="Thermometer [C]"() -> (w634:refnum<vi>)
    n430 = call "2_VisualizeModulePositioning2.vi"("Placement Monitor"=w768, "Calibrated positions of fiducials [mm]"=w774, "XYZ .NET Refnum in"=w691, "Axis Speeds"=w701, "Module fiducial marker"=w685, "N modules"=w689, "Sensor Pattern"=w633, "error in (no error)"=w700, "Templates path"=w773, "Calibration [um/pix]"=w770, "Current Build Phase"=w769, "Temperature"=w634, "Module #"=w707, "Placement tolerance [um]"="Placement tolerance [um]", "Module Report"=w772, "Base notes"=w658, "Reports path"=w664) -> ("Recalibrated??"=w651:bool, "XYZ .NET Refnum out"=w657:refnum<k24>, "error out"=w654:errorcluster)  [unwired: 8 in]
    n431 = Not(x=w651) -> (.not. x?=w655:bool)
    n432 = case shown="True" w651 {
      tunnel: [w775 w776] -> w653
      tunnel: w654 -> [w775 w776]
      frame False {
      }
      frame True {
        w777 = u16 2 items=["Bus Tape", "Tooling Pin", "Quick Calib"] ("Calibration Type")
        n433 = local write "Calibration Type"(w777) -> ()
      }
    }
  }
  n434 = property on="Tape Type" class="Enum (strict)"(error in=w71) -> (error out=w148:errorcluster, "Strings []"=w182:string[], "Value"=w144:T5)  [unwired: 1 in, 1 out]
  n435 = property on="Mounted?" class="Clust (strict)"(error in=w71, "Color"=u32 1089280) -> (error out=w132:errorcluster)  [unwired: 1 in, 1 out]
  n436 = Index Array(array=w182, index=w144) -> (element=w181:string)
  n437 = Concatenate Strings(w181, " stave side complete! " ("Current Build Phase")) -> (w179:string)
  n438 = property on="Current Build Phase" class="Str"(error in=w148, "Value"=w179) -> (error out=w133:errorcluster)  [unwired: 1 in, 1 out]
  n439 = Merge Errors(w69, w133, w132) -> (w131:errorcluster)
  n440 = property on="Tape Type" class="Enum (strict)"(error in=w131) -> (error out=w149:errorcluster, "Strings []"=w184:string[], "Value"=w143:T5)  [unwired: 1 in, 1 out]
  n441 = Index Array(array=w184, index=w143) -> (element=w185:string)
  n442 = Concatenate Strings(w185, " stave side survey in progress... " ("Current Build Phase")) -> (w183:string)
  n443 = property on="Current Build Phase" class="Str"(error in=w149, "Value"=w183) -> (error out=w81:errorcluster)  [unwired: 1 in, 1 out]
  n444 = property on="Axis Speeds [mm/s]" class="Clust (strict)"(error in=w81) -> (error out=w80:errorcluster, "Value"=w85:cluster{"X":dbl, "Y":dbl, "Z":dbl})  [unwired: 1 in, 1 out]
  n445 = property on="Before curing" class="Bool (strict)"(error in=w80, "Value"=w187) -> (error out=w89:errorcluster)  [unwired: 1 in, 1 out]
  n446 = local read "double( Time, Temp )"() -> (w83:dbl[])
  n447 = local read "Current field of view"() -> (w84:T23)
  n448 = local read "Reports path"() -> (w93:path)
  n449 = property on="Tape Type" class="Enum (strict)"(error in=w89) -> (error out=w87:errorcluster, "Strings []"=w193:string[], "Value"=w142:T5)  [unwired: 1 in, 1 out]
  n450 = call "0_StaveSurvey.vi"("Folder name for survey results"="AfterCure", "Axes Speeds [mm/s]"=w85, "Records directory"=w93, "error in (no error)"=w87, "double( Time, Temp )"=w83, "Most recently collected image"=w84, "XYZ Stage .NET Refnum in"=w70) -> ("Error report"=w86:errorcluster, "XYZ Stage .NET Refnum out"=w91:refnum<k24>)  [unwired: 3 in]
  n451 = Index Array(array=w193, index=w142) -> (element=w192:string)
  n452 = property on="After curing" class="Bool (strict)"(error in=w86, "Value"=w187) -> (error out=w88:errorcluster)  [unwired: 1 in, 1 out]
  n453 = Concatenate Strings(w192, " stave side complete! " ("Current Build Phase")) -> (w190:string)
  n454 = property on="Current Build Phase" class="Str"(error in=w88, "Value"=w190) -> (error out=w188:errorcluster)  [unwired: 1 in, 1 out]
  n455 = property on="Surveyed?" class="Clust (strict)"(error in=w188, "Color"=u32 1089280) -> (error out=w90:errorcluster)  [unwired: 1 in, 1 out]
  n456 = call "DisableMultiple.vi"("error in (no error)"=w90, "axis names"=string[] ["X", "Y", "Z"], "controller in"=w91) -> ("error out"=w98:errorcluster, "controller out"=w97:refnum<k24>)  [unwired: 7 in]
  n457 = call "Disconnect.vi"("error in (no error)"=w98, "controller"=w97) -> ("error out"=w82:errorcluster)  [unwired: 9 in]
  n458 = local write "Program Errors"(w82) -> ()
  "Calibration Results" <- T28 {"Camera calibration results"={"Calibration [um/pix]"=0.0, "Working distance to stave [mm]"=0.0, "Calib uncertainty [um/pix]"=0.0, "WD Uncertainty [mm]"=0.0}, "Stave basis calibration results"={"Angle, stave & xyz stage [rad]"=0.0, "Calibrated stave origin (X,Y) [mm]"=[0.0, 0.0]}} ("Calibration Results")
  "Module Progress Report" <- T3 [] ("Module Progress Report")
  "BUILD STAVE: STATUS REPORT" <- w52
  "Image Collection Progress" <- u8 0 ("Cam Calib Image\nCollection Status")
